vi "UHR-Fleezers Control (host) - 10.6.vi"() -> ()   [LabVIEW 2010] (continued)
    n794 = call <vilib>:"Mean.vi"("X"=w1127) -> ("mean"=w1106:dbl)  [unwired: 1 out]
    "T1 X" <- w1106
    n795 = Add(x=w1128, y=w1129) -> (x+y=w1130:dbl[])
    n796 = Bundle By Name(cluster=w1162, "Y"=w1124) -> (w1092:waveform(dbl))
    "Bead Separation" <- w1092
    n797 = Divide(x=w1130, y=2.0) -> (x/y=→"Vec Mean of T1 T2":dbl[])
    n798 = case shown="True" w1139 {
      tunnel: w1181 -> [_ w2041]
      tunnel: w1180 -> [_ w2040]
      tunnel: w1179 -> [_ w2039]
      tunnel: w1176 -> [_ w2038]
      tunnel: w1101 -> [_ w2037]
      frame False {
      }
      frame True {
        n799 = property on="Force" class="WFChart (strict)"("YScale.NameLbl.Text"=w2041) -> ()  [unwired: 2 in, 2 out]
        n800 = property on="T2 X" class="DigNum (strict)"("Caption.Text"=w2039) -> ()  [unwired: 2 in, 2 out]
        n801 = property on="T1 X" class="DigNum (strict)"("Caption.Text"=w2040) -> ()  [unwired: 2 in, 2 out]
        n802 = property on="Mean" class="DigNum (strict)"("Caption.Text"=w2038) -> ()  [unwired: 2 in, 2 out]
        n803 = property on="Difference" class="DigNum (strict)"("Caption.Text"=w2037) -> ()  [unwired: 2 in, 2 out]
      }
    }
    n804 = local read "Tether"() -> (w1133:bool)
    n805 = Absolute Value(x=w1106) -> (abs(x)=w1103:dbl)
    n806 = Absolute Value(x=w1105) -> (abs(x)=w1102:dbl)
    n807 = Add(x=w1103, y=w1102) -> (x+y=w1178:dbl)
    n808 = Subtract(x=w1103, y=w1102) -> (x-y=→"Difference":dbl)
    n809 = feedback #18(w1124) -> (w1123:dbl[])
    n810 = Divide(x=w1178, y=2.0) -> (x/y=w1132:dbl)
    "Mean" <- w1132
    n811 = case shown="True" w1133 {
      tunnel: w1132 -> [_ w1582]
      frame False {
      }
      frame True {
        n812 = Greater?(x="Lost Tether Alarm Threshold (pN)", y=w1582) -> (0:w1580:bool)
        n813 = case shown="True" w1580 {
          frame False {
          }
          frame True {
            n814 = flat-sequence {
              frame #0 {
                # "stop only if saving"
                n815 = local read "Saving..."() -> (w1595:bool)
                n816 = And(x=w1595, y="TA Cancel Save?") -> (x .and. y?=w1594:bool)
                n817 = local write "Stop Saving"(w1594) -> ()
              }
              frame #1 {
                n818 = case shown="True" "TA Green Off?" {
                  frame False {
                  }
                  frame True {
                    w1598 = FALSE ("Fl. Triggered...")
                    n819 = local write "Fl. Triggered..."(w1598) -> ()
                    n820 = property on="Green Laser ON/Interlacing" class="Bool (strict)"("Val(Sgnl)"=w1598) -> ()  [unwired: 2 in, 2 out]
                  }
                }
              }
            }
            n821 = local read "Time tether formed"() -> (w1589:timestamp)
            n822 = Get Date/Time In Seconds() -> (seconds since 1Jan1904=w1590:timestamp)
            n823 = Subtract(x=w1590, y=w1589) -> (x-y=w1588:dbl)
            n824 = Number To Decimal String(number=w1588) -> (decimal integer string=w1585:string)  [unwired: 1 out]
            n825 = local read "Messages"() -> (w1592:string)
            n826 = call <vilib>:"Beep.vi"() -> ()  [unwired: 3 in, 9 out]
            n827 = Concatenate Strings("Lost tether (" ("Message to add"), w1585, " s)." ("string")) -> (w1587:string)
            n828 = local write "Tether"(FALSE ("Tether")) -> ()
            n829 = call "Update messages.vi"("Message to add"=w1587, "Old message string"=w1592) -> ("New message string"=w1591:string)
            n830 = local write "Messages"(w1591) -> ()
            n831 = property on="Trap Pos. FB ON" class="Bool (strict)"("Val(Sgnl)"=FALSE ("Value (Signaling)")) -> ()  [unwired: 2 in, 2 out]
          }
        }
      }
    }
    n832 = Build Array (concatenate)(w1124, w1123) -> (w1122:dbl[])
    n833 = Split 1D Array(array=w1122, index=w1004) -> (first subarray=w1118:dbl[])  [unwired: 1 out]
    n834 = feedback-in #18(w1118) -> ()
    n835 = call <vilib>:"Mean.vi"("X"=w1118) -> ("mean"=w1117:dbl)  [unwired: 1 out]
    "Bead Mean (nm)" <- w1117
    n836 = Subtract(x=w1118, y=w1117) -> (x-y=w1116:dbl[])
    n837 = Square(x=w1116) -> (x^2=w1115:dbl[])
    n838 = call <vilib>:"Mean.vi"("X"=w1115) -> ("mean"=w1114:dbl)  [unwired: 1 out]
    n839 = Square Root(x=w1114) -> (sqrt(x)=w1113:dbl)
    n840 = Multiply(x=10.0, y=w1113) -> (x*y=→"RMS (Ang)":dbl)
    n841 = xnode "Read/Write Control"("FPGA VI Reference In"=w1154, "error in"=w1153) -> ("FPGA VI Reference Out"=w1270:T20, "error out"=w1264:errorcluster, "AI2 Y Sum Set 1"=w1260:i16, "AI2 Y Sum Set 2"=w1259:i16, "AI1 X Set 1"=w1038:fxp<+/-,16,1>, "AI1 X Set 2"=w1037:fxp<+/-,16,1>, "Trap Pos FB Int Signal"=→"Trap Pos FB Int Signal":fxp<+/-,24,9>, "Trap Pos FB Int-Norm Signal"=→"Trap Pos FB Int-Norm Signal":fxp<+/-,16,1>, "Trap Pos FB Action"=w1031:i64, "Scanning"=→"AOD Scanning":bool, "Scan I"=→"AOD Scan I":u64, "Scanning MCL"=w1262:bool, "Scan I (MCL)"=→"MCL Scan I":u64, "Green FB Signals"=w1199:T38)  [unwired: 1 out]
    "MCL Scanning" <- w1262
    "Trap Pos FB Action" <- w1031
    n842 = local read "AI2 (V)"() -> (w1261:cluster{"Set 1":dbl, "Set 2":dbl})
    n843 = Bundle By Name(cluster=w1261, "Set 1"=w1260, "Set 2"=w1259) -> (w1257:cluster{"Set 1":dbl, "Set 2":dbl})
    n844 = Divide(x=w1031, y=327.67) -> (x/y=→"Action (%)":dbl)
    n845 = local read "Trap X (AI1)"() -> (w1051:T10)
    n846 = Divide(x=w1257, y=3276.7) -> (x/y=w1256:cluster{"Set 1":dbl, "Set 2":dbl})
    n847 = local write "AI2 (V)"(w1256) -> ()
    n848 = Bundle(cluster=w1051, "Trap 1"=w1038, "Trap 2"=w1037) -> (→"Trap X (AI1)":T10)
    n849 = Divide(x=w1199, y=3276.7) -> (x/y=w1195:T46)
    n850 = Unbundle By Name(w1195) -> ("Green FB Ch 0"=w1198:dbl, "Green FB Ch 1"=w1197:dbl, "Green FB Ch 2"=w1196:dbl)
    n851 = Divide(x=w1198, y=w1196) -> (x/y=w1194:dbl)
    n852 = Divide(x=w1197, y=w1196) -> (x/y=w1193:dbl)
    n853 = flat-sequence "To save data" {
      tunnel: [w3898] -> w1281
      tunnel: [w3899] -> w1280
      tunnel: w1230 -> [w3892]
      tunnel: w1120 -> [w3896]
      tunnel: ["Save Calibration"] -> w1253
      tunnel: w1250 -> [w3895]
      tunnel: [w3888] -> w1249
      tunnel: [w3885] -> w1248
      tunnel: [w3882] -> w1247
      tunnel: w1229 -> [w3884]
      tunnel: w1137 -> [w3878]
      tunnel: [w3878] -> w1136
      tunnel: ["Start Saving"] -> w1094
      tunnel: [w3872] -> w1020
      tunnel: [w3871] -> w1019
      tunnel: w1281 -> [w4133]
      tunnel: w1280 -> [w4132]
      tunnel: w1021 -> [w4131]
      tunnel: w1253 -> [w4130]
      tunnel: w1249 -> [w4128]
      tunnel: w1248 -> [w4127]
      tunnel: w1247 -> [w4126]
      tunnel: w1107 -> [w4125]
      tunnel: w1146 -> [w4124]
      tunnel: w1136 -> [w4123]
      tunnel: w1094 -> [w4122]
      tunnel: w1092 -> [w4121]
      tunnel: w1068 -> [w4120]
      tunnel: w1020 -> [w4119]
      tunnel: w1019 -> [w4118]
      tunnel: w1018 -> [w4117]
      frame #0 {
        n854 = Or(x="Save N Sets", y="Start Saving") -> (x .or. y?=w3879:bool)
        n855 = To Double Precision Float(number=w3895) -> (double precision float=w3889:dbl)
        n856 = Build Array(w3879, "Save Calibration", w3892, w3884) -> (w3894:bool[])
        n857 = Compound Arithmetic op=OR("Save Calibration", w3892, w3879, w3884) -> (w3897:bool)
        n858 = Boolean Array To Number(Boolean array=w3894) -> (number=w3891:u32)
        n859 = feedback #19(FALSE ("Save APD Data\nwith Trap Data")) -> (w3873:bool)
        n860 = feedback #20(refnum<k0> refnum) -> (w3900:refnum<file>)
        n861 = feedback #21(refnum<k0> refnum) -> (w3875:refnum<file>)
        n862 = feedback #22(FALSE ("Save APD Data\nwith Trap Data")) -> (w3883:bool)
        n863 = feedback #23(refnum<k0> refnum) -> (w3886:refnum<file>)
        n864 = feedback #24(0) -> (w3902:i32)
        n865 = feedback #25() -> (w3890:u32)  [unwired: 1 out]
        n866 = case shown="True" w3897 {
          tunnel: [w3909 1] -> w3898
          tunnel: w3902 -> [w3911 _]
          tunnel: [w3910 w3929] -> w3899
          tunnel: w3900 -> [w3910 _]
          tunnel: w3896 -> [_ w3949]
          tunnel: w3889 -> [_ w3947]
          tunnel: w3891 -> [_ w3950]
          tunnel: [w3908 w3928] -> w3888
          tunnel: w3890 -> [w3908 _]
          tunnel: [w3907 w3926] -> w3885
          tunnel: w3886 -> [w3907 _]
          tunnel: [w3906 w3925] -> w3882
          tunnel: w3883 -> [w3906 _]
          tunnel: "Start Saving" -> [_ w3923]
          tunnel: w3878 -> [_ w3922]
          tunnel: [w3905 w3913] -> w3871
          tunnel: w3875 -> [w3905 _]
          tunnel: [w3904 w3912] -> w3872
          tunnel: w3873 -> [w3904 _]
          frame False {
            n867 = Increment(x=w3911) -> (x+1=w3909:i32)
          }
          frame True {
            w3919 = FALSE ("Start Saving")
            w3924 = 9.0  # File Version
            w3932 = FALSE ("prepend array or string size? (T)")
            w3930 = T39."big-endian, network order" ("byte order (0:big-endian, network order)")
            # "write file headers"
            n868 = local read "BD 1 Frequency 1 (MHz)"() -> (w3946:dbl)
            n869 = local read "BD 2 Frequency 1 (MHz)"() -> (w3945:dbl)
            n870 = local read "BD 1 Frequency 2 (MHz)"() -> (w3944:dbl)
            n871 = local read "BD 2 Frequency 2 (MHz)"() -> (w3943:dbl)
            n872 = local read "BD 1 Frequency 3 (MHz)"() -> (w3942:dbl)
            n873 = local read "BD 2 Frequency 3 (MHz)"() -> (w3941:dbl)
            n874 = Array Size(array=w3922) -> (size(s)=w3921:i32)
            n875 = To Double Precision Float(number=w3921) -> (double precision float=w3920:dbl)
            n876 = local write "Save Calibration"(w3919) -> ()
            n877 = local write "Start Saving"(w3919) -> ()
            n878 = Build Array("Save APD Data\nwith Trap Data", "Save Trap Pos. Data") -> (w3916:bool[])
            n879 = Boolean Array To Number(Boolean array=w3916) -> (number=w3915:u32)
            n880 = Build Array(w3946, w3945, w3944, w3943, w3942, w3941) -> (w3940:dbl[])
            n881 = case shown="2" w3950 {
              tunnel: w3949 -> [w4021 w4041 w4057 w4095]
              tunnel: w3920 -> [w4026 w4048 w4077 w4114]
              tunnel: w3947 -> [w4025 w4047 w4076 w4113]
              tunnel: [w4022 w4043 w4068 w4105] -> w3938
              tunnel: [w4013 "Cal sets to save" w4058 w4096] -> w3928
              tunnel: w3940 -> [w4023 w4044 w4070 w4107]
              tunnel: "Save APD Data\nwith Trap Data" -> [w4020 _ w4054 w4093]
              tunnel: [w4020 w4035 w4054 w4093] -> w3925
              tunnel: w3924 -> [w4016 w4036 w4052 w4091]
              tunnel: w3923 -> [w4015 _ _ _]
              tunnel: [w4006 w4035 w4051 w4081] -> w3912
              tunnel: "Save Trap Pos. Data" -> [w4006 _ w4051 w4081]
              tunnel: w3915 -> [w4005 _ w4050 w4080]
              frame 1, Default {
                # "timeseries"
                n882 = case shown="True" "Profile" {
                  tunnel: [w4029 w4032] -> w4010
                  tunnel: [w4029 w4031] -> w4009
                  tunnel: [w4029 w4030] -> w4008
                  tunnel: [w4029 w4034] -> w4007
                  frame False {
                    w4029 = 0.0 ("f")
                  }
                  frame True {
                    n883 = local read "Current Position"() -> (w4033:dbl[])
                    n884 = local read "Y change (mm)"() -> (w4034:dbl)
                    n885 = call "subVI_explode3array.vi"("Array"=w4033) -> ("x"=w4032:dbl, "y"=w4031:dbl, "z"=w4030:dbl)  [unwired: 12 in]
                  }
                }
                n886 = local read "Save ave N"() -> (w4028:dbl)
                n887 = Multiply(x=w4028, y=w4021) -> (x*y=w4027:dbl)
                n888 = To Double Precision Float(number=w4005) -> (double precision float=w4019:dbl)
                n889 = Build Array(w4016, w4021, w4027, w4026, w4025, 0.0 ("f")) -> (w4024:dbl[])
                n890 = Build Array(w4019, w4010, w4009, w4008, w4007) -> (w4017:dbl[])
                n891 = Select(t=u32 4000000000, s=w4015, f="N sets to save") -> (s? t:f=w4013:u32)
                n892 = Build Array (concatenate)(w4024, w4023, w4017) -> (w4022:dbl[])
              }
              frame 2 {
                w4038 = 0.0 ("f")
                w4035 = FALSE ("Save APD Data\nwith Trap Data")
                # "calibration"
                n893 = Boolean To (0,1)(Boolean=w4035) -> (0, 1=w4040:i16)
                n894 = To Double Precision Float(number=w4040) -> (double precision float=w4039:dbl)
                n895 = Build Array(w4039, w4038, w4038, w4038, w4038) -> (w4037:dbl[])
                n896 = Build Array(w4036, w4041, w4041, w4048, w4047, 1.0 ("t")) -> (w4045:dbl[])
                n897 = Build Array (concatenate)(w4045, w4044, w4037) -> (w4043:dbl[])
                "Calibrating Trap..." <- TRUE ("Calibrating...")
              }
              frame 4 {
                w4055 = 0.0 ("f")
                # "scan dir (x/y = 0/1)"
                # "cycles/step"
                # "n scans (f/b)"
                # "steps"
                # "freq. range"
                # "AOD raster scan"
                n898 = local read "Number of F/B Scans (AOD)"() -> (w4062:u16)
                n899 = local read "Cycles/step (AOD)"() -> (w4064:u64)
                n900 = local read "Scan Range (MHz)"() -> (w4067:dbl)
                n901 = local read "Scan steps (AOD)"() -> (w4066:u64)
                n902 = local read "Scan BD"() -> (w4074:bool)
                n903 = local read "Save ave N"() -> (w4079:dbl)
                n904 = Boolean To (0,1)(Boolean=w4074) -> (0, 1=w4073:i16)
                n905 = To Double Precision Float(number=w4062) -> (double precision float=w4061:dbl)
                n906 = To Double Precision Float(number=w4066) -> (double precision float=w4065:dbl)
                n907 = To Double Precision Float(number=w4064) -> (double precision float=w4063:dbl)
                n908 = To Double Precision Float(number=w4073) -> (double precision float=w4072:dbl)
                n909 = Multiply(x=w4079, y=w4057) -> (x*y=w4078:dbl)
                n910 = To Double Precision Float(number=w4050) -> (double precision float=w4056:dbl)
                n911 = Build Array(w4056, w4055, w4055, w4055, w4055) -> (w4053:dbl[])
                n912 = local read "N sets should be saved"() -> (w4059:dbl)
                n913 = Build Array(w4072, w4067, w4065, w4063, w4061) -> (w4069:dbl[])
                n914 = Build Array(w4052, w4057, w4078, w4077, w4076, 2.0 ("t")) -> (w4071:dbl[])
                n915 = Round Toward +Infinity(x=w4059) -> (ceil(x): smallest int >= x=w4060:dbl)
                n916 = Build Array (concatenate)(w4071, w4070, w4053, w4069) -> (w4068:dbl[])
                n917 = To Unsigned Long Integer(number=w4060) -> (unsigned 32bit integer=w4058:u32)
              }
              frame 8 {
                w4088 = 0.0 ("f")
                # "MCL raster scan"
                n918 = local read "Number of scans (MCL)"() -> (w4083:u64)
                n919 = local read "Scan lines (y)"() -> (w4082:u64)
                n920 = local read "2D or 1D Scan"() -> (w4085:bool)
                n921 = local read "Scan Range (V)\n(of steps)"() -> (w4104:dbl)
                n922 = local read "Fast Scan Dir"() -> (w4111:bool)
                n923 = local read "Cycles/step (MCL)"() -> (w4101:u64)
                n924 = local read "Scan steps (MCL)"() -> (w4103:u64)
                n925 = Select(t=w4082, s=w4085, f=w4083) -> (s? t:f=w4084:u64)
                n926 = Boolean To (0,1)(Boolean=w4085) -> (0, 1=w4087:i16)
                n927 = local read "Save ave N"() -> (w4116:dbl)
                n928 = local read "Initial X"() -> (w4090:dbl)
                n929 = local read "Initial Y"() -> (w4089:dbl)
                n930 = To Double Precision Float(number=w4087) -> (double precision float=w4086:dbl)
                n931 = Boolean To (0,1)(Boolean=w4111) -> (0, 1=w4110:i16)
                n932 = To Double Precision Float(number=w4084) -> (double precision float=w4099:dbl)
                n933 = To Double Precision Float(number=w4103) -> (double precision float=w4102:dbl)
                n934 = To Double Precision Float(number=w4101) -> (double precision float=w4100:dbl)
                n935 = To Double Precision Float(number=w4110) -> (double precision float=w4109:dbl)
                n936 = Multiply(x=w4116, y=w4095) -> (x*y=w4115:dbl)
                n937 = To Double Precision Float(number=w4080) -> (double precision float=w4094:dbl)
                n938 = local read "N sets should be saved (MCL)"() -> (w4097:dbl)
                n939 = Build Array(w4094, w4086, w4088, w4088, w4088) -> (w4092:dbl[])
                n940 = Build Array(w4109, w4104, w4102, w4100, w4099, w4090, w4089) -> (w4106:dbl[])
                n941 = Build Array(w4091, w4095, w4115, w4114, w4113, 3.0 ("t")) -> (w4108:dbl[])
                n942 = Round Toward +Infinity(x=w4097) -> (ceil(x): smallest int >= x=w4098:dbl)
                n943 = Build Array (concatenate)(w4108, w4107, w4092, w4106) -> (w4105:dbl[])
                n944 = To Unsigned Long Integer(number=w4098) -> (unsigned 32bit integer=w4096:u32)
              }
            }
            n945 = local read "Index"() -> (w3955:dbl)
            n946 = call "Create new save file.vi"("Insert"="", "Ext"=".dat", "Index In"=w3955) -> ("Path Out"=w3914:path, "Index Out"=w3927:dbl)
            n947 = local write "Save file name"(w3914) -> ()
            n948 = local write "Index"(w3927) -> ()
            n949 = local write "Save index"(w3927) -> ()
            n950 = Array Size(array=w3938) -> (size(s)=w3939:i32)
            n951 = Open/Create/Replace File(file path (use dialog)=w3914, operation (0:open)=T25."create", access (0:read/write)=enum16{"read/write", "read-only", "write-only"}."write-only") -> (refnum out=w3952:refnum<file>)  [unwired: 1 in, 4 out]
            n952 = local write "Saving..."(TRUE ("Saving...")) -> ()
            n953 = To Double Precision Float(number=w3939) -> (double precision float=w3937:dbl)
            n954 = String Length(string="Comment (data description)") -> (length=w3935:i32)
            n955 = To Double Precision Float(number=w3935) -> (double precision float=w3934:dbl)
            n956 = Deny Access(7:w3952) -> (3:w3951:refnum<file>)  [unwired: 1 in, 2 out]
            n957 = Build Array (concatenate)(w3937, w3938, w3934) -> (w3936:dbl[])
            n958 = case "If fluorescence data to be saved" shown="False" w3925 {
              tunnel: w3914 -> [_ w4004]
              tunnel: [refnum<k0> refnum w3984] -> w3926
              frame False {
              }
              frame True {
                w3983 = 0.0
                n959 = local read "APD Integration Time (s)"() -> (w3989:dbl)
                n960 = local read "N APD Samp/step"() -> (w3982:dbl)
                n961 = Path To String(path=w4004) -> (string=w4003:string)
                n962 = String Length(string=w4003) -> (length=w4002:i32)
                n963 = Subtract(x=w4002, y=4) -> (x-y=w4000:i32)
                n964 = String Subset(string=w4003, length (rest)=w4000) -> (substring=w3999:string)  [unwired: 1 out]
                n965 = Build Array(w3989, w3982, w3983, w3983, w3983, w3983, w3983, w3983) -> (w3986:dbl[])
                n966 = Concatenate Strings(w3999, "_fl.dat" ("string")) -> (w3997:string)
                n967 = Array Size(array=w3986) -> (size(s)=w3988:i32)
                n968 = String To Path(string=w3997) -> (path=w3993:path)
                n969 = Open/Create/Replace File(file path (use dialog)=w3993, operation (0:open)=T25."create", access (0:read/write)=enum16{"read/write", "read-only", "write-only"}."write-only") -> (refnum out=w3994:refnum<file>)  [unwired: 1 in, 4 out]
                n970 = Deny Access(7:w3994) -> (3:w3990:refnum<file>)  [unwired: 1 in, 2 out]
                n971 = To Double Precision Float(number=w3988) -> (double precision float=w3987:dbl)
                n972 = Build Array (concatenate)(w3987, w3986) -> (w3985:dbl[])
                n973 = Write to Binary File(file (use dialog)=w3990, data=w3985, 5:FALSE ("prepend array or string size? (T)"), 9:T39."big-endian, network order" ("byte order (0:big-endian, network order)")) -> (refnum out=w3984:refnum<file>)  [unwired: 1 in, 3 out]
              }
            }
            n974 = case shown="True" w3912 {
              tunnel: w3914 -> [_ w3966]
              tunnel: [refnum<k0> refnum w3965] -> w3913
              frame False {
              }
              frame True {
                w3961 = 0.0 ("element")
                n975 = Path To String(path=w3966) -> (string=w3980:string)
                n976 = Build Array(w3961, w3961, w3961, w3961, w3961, w3961, w3961, w3961) -> (w3962:dbl[])
                n977 = String Length(string=w3980) -> (length=w3979:i32)
                n978 = Subtract(x=w3979, y=4) -> (x-y=w3977:i32)
                n979 = Array Size(array=w3962) -> (size(s)=w3964:i32)
                n980 = String Subset(string=w3980, length (rest)=w3977) -> (substring=w3976:string)  [unwired: 1 out]
                n981 = To Double Precision Float(number=w3964) -> (double precision float=w3963:dbl)
                n982 = Concatenate Strings(w3976, "_pos.dat" ("string")) -> (w3974:string)
                n983 = Build Array (concatenate)(w3963, w3962) -> (w3960:dbl[])
                n984 = String To Path(string=w3974) -> (path=w3970:path)
                n985 = Open/Create/Replace File(file path (use dialog)=w3970, operation (0:open)=T25."create", access (0:read/write)=enum16{"read/write", "read-only", "write-only"}."write-only") -> (refnum out=w3971:refnum<file>)  [unwired: 1 in, 4 out]
                n986 = Deny Access(7:w3971) -> (3:w3967:refnum<file>)  [unwired: 1 in, 2 out]
                n987 = Write to Binary File(file (use dialog)=w3967, data=w3960, 5:FALSE ("prepend array or string size? (T)"), 9:T39."big-endian, network order" ("byte order (0:big-endian, network order)")) -> (refnum out=w3965:refnum<file>)  [unwired: 1 in, 3 out]
              }
            }
            n988 = Write to Binary File(file (use dialog)=w3951, data=w3936, 5:w3932, 9:w3930) -> (refnum out=w3933:refnum<file>)  [unwired: 1 in, 3 out]
            n989 = Write to Binary File(file (use dialog)=w3933, data="Comment (data description)", 5:w3932, 9:w3930) -> (refnum out=w3929:refnum<file>)  [unwired: 1 in, 3 out]
          }
        }
        n990 = feedback-in #19(w3872) -> ()
        n991 = feedback-in #20(w3899) -> ()
        n992 = feedback-in #21(w3871) -> ()
        n993 = feedback-in #22(w3882) -> ()
        n994 = feedback-in #23(w3885) -> ()
        n995 = feedback-in #24(w3898) -> ()
        n996 = feedback-in #25(w3888) -> ()
      }
      frame #1 {
        n997 = local read "Saving..."() -> (w4129:bool)
        n998 = case shown="True" w4129 {
          tunnel: w4133 -> [_ w4143]
          tunnel: w4132 -> [_ w4157]
          tunnel: w4131 -> [_ w4153]
          tunnel: w4130 -> [_ w4152]
          tunnel: w4128 -> [_ w4151]
          tunnel: w4127 -> [_ w4146]
          tunnel: w4126 -> [_ w4145]
          tunnel: w4125 -> [_ w4144]
          tunnel: w4124 -> [_ w4142]
          tunnel: w4123 -> [_ w4140]
          tunnel: w4122 -> [_ w4139]
          tunnel: w4121 -> [_ w4138]
          tunnel: w4120 -> [_ w4137]
          tunnel: w4119 -> [_ w4136]
          tunnel: w4118 -> [_ w4135]
          tunnel: w4117 -> [_ w4134]
          frame False {
          }
          frame True {
            n999 = Multiply(x=w4143, y=w4142) -> (x*y=→"Time (s)":dbl)
            n1000 = Less Or Equal?(x=w4143, y=w4151) -> (x <= y?=w4155:bool)
            n1001 = Or(x="Stop Saving", y="Abort save 2") -> (x .or. y?=w4147:bool)
            n1002 = Not(x=w4147) -> (.not. x?=w4156:bool)
            n1003 = And(x=w4155, y=w4156) -> (x .and. y?=w4154:bool)
            n1004 = case shown="True" w4154 {
              tunnel: w4157 -> [w4164 w4232]
              tunnel: [0.0 w4235] -> w4150
              tunnel: w4143 -> [_ w4233]
              tunnel: w4151 -> [_ w4234]
              tunnel: w4153 -> [_ w4229]
              tunnel: w4152 -> [_ _]
              tunnel: w4146 -> [w4162 w4222]
              tunnel: w4145 -> [w4161 w4223]
              tunnel: w4144 -> [_ w4221]
              tunnel: w4140 -> [_ w4220]
              tunnel: w4139 -> [_ w4174]
              tunnel: w4138 -> [_ w4213]
              tunnel: w4137 -> [_ w4191]
              tunnel: w4136 -> [w4158 w4172]
              tunnel: w4135 -> [w4159 w4171]
              tunnel: w4134 -> [_ w4168]
              frame False {
                w4160 = FALSE
                n1005 = Close File(refnum=w4164) -> ()  [unwired: 1 in, 2 out]
                n1006 = case shown="True" w4161 {
                  tunnel: w4162 -> [_ w4166]
                  frame False {
                  }
                  frame True {
                    n1007 = Close File(refnum=w4166) -> ()  [unwired: 1 in, 2 out]
                  }
                }
                n1008 = case shown="True" w4158 {
                  tunnel: w4159 -> [_ w4165]
                  frame False {
                  }
                  frame True {
                    n1009 = Close File(refnum=w4165) -> ()  [unwired: 1 in, 2 out]
                  }
                }
                n1010 = local write "Raster Scanning..."(w4160) -> ()
                n1011 = local write "Calibrating Trap..."(w4160) -> ()
                n1012 = call <vilib>:"Beep.vi"() -> ()  [unwired: 3 in, 9 out]
                n1013 = local write "Stop Saving"(w4160) -> ()
                "Saving..." <- w4160
              }
              frame True {
                n1014 = local read "Calibrating Trap..."() -> (w4224:bool)
                n1015 = case "Write fl. data" shown="True" w4223 {
                  tunnel: w4222 -> [_ w4258]
                  tunnel: w4221 -> [_ w4257]
                  frame False {
                  }
                  frame True {
                    n1016 = Write to Binary File(file (use dialog)=w4258, data=w4257, 5:FALSE ("prepend array or string size? (T)"), 9:T39."big-endian, network order" ("byte order (0:big-endian, network order)")) -> ()  [unwired: 1 in, 4 out]
                  }
                }
                n1017 = Greater?(x="Save ave N", y=1.0) -> (0:w4227:bool)
                n1018 = Not(x=w4224) -> (.not. x?=w4226:bool)
                n1019 = And(x=w4226, y=w4227) -> (x .and. y?=w4169:bool)
                n1020 = case shown="True" w4169 {
                  tunnel: w4168 -> [w4238 w4249]
                  tunnel: [w4238 w4241] -> w4167
                  tunnel: "Save ave N" -> [_ w4242]
                  frame False {
                  }
                  frame True {
                    w4239 = 2 ("dimension size")
                    n1021 = Array Size(array=w4249) -> (size(s)=w4243:i32)
                    n1022 = Divide(x=w4243, y=w4239) -> (x/y=w4247:dbl)
                    n1023 = Reshape Array(w4249, w4247, w4239) -> (w4248:u64[][])
                    n1024 = Transpose 2D Array(2D array=w4248) -> (transposed array=w4246:u64[][])
                    n1025 = for {
                      tunnel: w4246 -> [w4251] mode=indexing
                      tunnel: [w4250] -> w4240 mode=indexing
                      tunnel: w4242 -> [w4252]
                      workers-P: _ -> [_]
                      n1026 = call "downsample 1D array - U64.vi"("Ave N"=w4252, "Array In"=w4251) -> ("Array Out"=w4250:u64[])  [unwired: 1 in]
                    }
                    n1027 = Transpose 2D Array(2D array=w4240) -> (transposed array=w4245:u64[][])
                    n1028 = Divide(x=w4243, y=w4242) -> (x/y=w4244:dbl)
                    n1029 = Reshape Array(w4245, w4244) -> (w4241:u64[])
                  }
                }
                n1030 = case shown="True" w4169 {
                  tunnel: w4229 -> [w4261 w4273]
                  tunnel: [w4261 w4262] -> w4225
                  tunnel: "Save ave N" -> [_ w4266]
                  tunnel: w4220 -> [_ w4265]
                  frame False {
                    # "don't downsample data for trap calibration"
                  }
                  frame True {
                    n1031 = Array Size(array=w4273) -> (size(s)=w4267:i32)
                    n1032 = Array Size(array=w4265) -> (size(s)=w4264:i32)
                    n1033 = Divide(x=w4267, y=w4264) -> (x/y=w4271:dbl)
                    n1034 = Reshape Array(w4273, w4271, w4264) -> (w4272:i16[][])
                    n1035 = Transpose 2D Array(2D array=w4272) -> (transposed array=w4270:i16[][])
                    n1036 = for {
                      tunnel: w4270 -> [w4276] mode=indexing
                      tunnel: [w4275] -> w4263 mode=indexing
                      tunnel: w4266 -> [w4274]
                      workers-P: _ -> [_]
                      n1037 = call "downsample 1D array - I16.vi"("Ave N"=w4274, "Array In"=w4276) -> ("Array Out"=w4275:i16[])  [unwired: 1 out]
                    }
                    n1038 = Transpose 2D Array(2D array=w4263) -> (transposed array=w4269:i16[][])
                    n1039 = Divide(x=w4267, y=w4266) -> (x/y=w4268:dbl)
                    n1040 = Reshape Array(w4269, w4268) -> (w4262:i16[])
                  }
                }
                n1041 = Index Array(array=w4191, index=1) -> (element=w4194:waveform(dbl))
                n1042 = Index Array(array=w4191, index=0) -> (element=w4196:waveform(dbl))
                n1043 = Unbundle By Name(w4194) -> ("Y"=w4198:dbl[])
                n1044 = Unbundle By Name(w4196) -> ("Y"=w4206:dbl[])
                n1045 = case "Write trap pos. data" shown="True" w4172 {
                  tunnel: w4171 -> [_ w4254]
                  tunnel: w4167 -> [_ w4253]
                  frame False {
                  }
                  frame True {
                    n1046 = Write to Binary File(file (use dialog)=w4254, data=w4253, 5:FALSE ("prepend array or string size? (T)"), 9:T39."big-endian, network order" ("byte order (0:big-endian, network order)")) -> ()  [unwired: 1 in, 4 out]
                  }
                }
                n1047 = Write to Binary File(file (use dialog)=w4232, data=w4225, 5:FALSE ("prepend array or string size? (T)"), 9:T39."big-endian, network order" ("byte order (0:big-endian, network order)")) -> ()  [unwired: 1 in, 4 out]
                n1048 = feedback #26(w4198) -> (w4200:dbl[])
                n1049 = Build Array (concatenate)(w4200, w4198) -> (w4199:dbl[])
                n1050 = Select(t=w4198, s=w4174, f=w4199) -> (s? t:f=w4184:dbl[])
                n1051 = feedback-in #26(w4184) -> ()
                n1052 = feedback #27(w4206) -> (w4219:dbl[])
                n1053 = Build Array (concatenate)(w4219, w4206) -> (w4218:dbl[])
                n1054 = Select(t=w4206, s=w4174, f=w4218) -> (s? t:f=w4193:dbl[])
                n1055 = feedback-in #27(w4193) -> ()
                n1056 = Divide(x=w4233, y=w4234) -> (x/y=w4236:dbl)
                n1057 = Multiply(x=w4236, y=100.0) -> (x*y=w4235:dbl)
                n1058 = Build Array(w4193, w4184) -> (→"Saved APD":dbl[][])
                n1059 = Array Size(array=w4193) -> (size(s)=w4211:i32)
                n1060 = Unbundle By Name(w4213) -> ("Y"=w4217:dbl[])
                n1061 = Subtract(x=w4211, y="N pts to average") -> (x-y=w4187:i32)
                n1062 = Multiply(x="N pts to average", y=u16 2) -> (x*y=w4188:u16)
                n1063 = Subtract(x=w4211, y=w4188) -> (x-y=w4186:i32)
                n1064 = feedback #28(w4217) -> (w4216:dbl[])
                n1065 = Build Array (concatenate)(w4216, w4217) -> (w4215:dbl[])
                n1066 = Select(t=w4217, s=w4174, f=w4215) -> (s? t:f=w4214:dbl[])
                "Trap Delta Graph" <- w4214
                n1067 = feedback-in #28(w4214) -> ()
                n1068 = Array Subset(array=w4193, index=w4187, length="N pts to average") -> (w4210:dbl[])
                n1069 = Array Subset(array=w4193, index=w4186, length="N pts to average") -> (w4209:dbl[])
                n1070 = Array Subset(array=w4184, index=w4187, length="N pts to average") -> (w4190:dbl[])
                n1071 = Array Subset(array=w4184, index=w4186, length="N pts to average") -> (w4189:dbl[])
                n1072 = call <vilib>:"Mean.vi"("X"=w4210) -> ("mean"=w4208:dbl)  [unwired: 1 out]
                n1073 = call <vilib>:"Mean.vi"("X"=w4190) -> ("mean"=w4183:dbl)  [unwired: 1 out]
                n1074 = call <vilib>:"Mean.vi"("X"=w4209) -> ("mean"=w4207:dbl)  [unwired: 1 out]
                n1075 = call <vilib>:"Mean.vi"("X"=w4189) -> ("mean"=w4182:dbl)  [unwired: 1 out]
                n1076 = Subtract(x=w4183, y=w4182) -> (x-y=w4173:dbl)
                "Delta Fl. 2" <- w4173
                n1077 = Subtract(x=w4208, y=w4207) -> (x-y=w4205:dbl)
                "Delta Fl. 1" <- w4205
                n1078 = Initialize Array(w4205, 1 ("dimension size")) -> (w4202:dbl[])
                n1079 = Initialize Array(w4173, 1 ("dimension size")) -> (w4179:dbl[])
                n1080 = feedback #29(w4202) -> (w4203:dbl[])
                n1081 = Build Array (concatenate)(w4203, w4202) -> (w4201:dbl[])
                n1082 = feedback #30(w4179) -> (w4180:dbl[])
                n1083 = Build Array (concatenate)(w4180, w4179) -> (w4178:dbl[])
                n1084 = Select(t=w4202, s=w4174, f=w4201) -> (s? t:f=w4177:dbl[])
                n1085 = feedback-in #29(w4177) -> ()
                n1086 = Select(t=w4179, s=w4174, f=w4178) -> (s? t:f=w4176:dbl[])
                n1087 = feedback-in #30(w4176) -> ()
                n1088 = Build Array(w4177, w4176) -> (→"Save APD Deriv":dbl[][])
              }
            }
            "Progress" <- w4150
            "Progress 2" <- w4150
          }
        }
      }
    }
    n1089 = Bundle By Name(cluster=w1195, "Green FB Ch 0"=w1194, "Green FB Ch 1"=w1193) -> (w1175:T46)
    "Green FB Signals (V)" <- w1175
    n1090 = Unbundle By Name(w1175) -> ("Green FB Ch 2"=→"Green FB Plot":dbl)
    n1091 = local read "wait to reset values"() -> (w1265:bool)
    n1092 = Not(x=w1262) -> (.not. x?=w1266:bool)
    n1093 = And(x=w1266, y=w1265) -> (x .and. y?=w1267:bool)
    n1094 = case "Part of MCL raster scanning: returns to initial positions after scan done" shown="True" w1267 {
      tunnel: w1270 -> [w2867 w2874]
      tunnel: [w2867 w2873] -> w1269
      tunnel: w1264 -> [w2866 w2872]
      tunnel: [w2866 w2871] -> w1263
      frame False {
      }
      frame True {
        w2882 = 10.0 ("y")
        w2881 = 32767.0 ("y")
        # "to return scan values\nafter a synchronous \nAOM scan"
        n1095 = local read "AO2"() -> (w2875:dbl)
        n1096 = local read "AO1"() -> (w2876:dbl)
        n1097 = local write "wait to reset values"(FALSE ("wait to reset values")) -> ()
        n1098 = Multiply(x=w2876, y=w2881) -> (x*y=w2878:dbl)
        n1099 = Multiply(x=w2875, y=w2881) -> (x*y=w2880:dbl)
        n1100 = Divide(x=w2878, y=w2882) -> (x/y=w2877:dbl)
        n1101 = Divide(x=w2880, y=w2882) -> (x/y=w2879:dbl)
        n1102 = To Word Integer(number=w2877) -> (16bit integer=w2883:i16)
        n1103 = To Word Integer(number=w2879) -> (16bit integer=w2884:i16)
        n1104 = local read "Total Counts (ticks)"() -> (w2868:u32)
        n1105 = xnode "Read/Write Control"("FPGA VI Reference In"=w2874, "error in"=w2872, "AO1"=w2883, "AO2"=w2884, "MCL count"=w2868) -> ("FPGA VI Reference Out"=w2873:T20, "error out"=w2871:errorcluster)
        n1106 = local read "Scan Range (V)\n(of steps)"() -> (w2869:dbl)
        n1107 = property on="Scan Range (V)\n(of steps)" class="DigNum (strict)"("Val(Sgnl)"=w2869) -> ()  [unwired: 2 in, 2 out]
      }
    }
    n1108 = node-c288() -> ()  [unwired: 2 out]
  }
  n1109 = node-c288(3 ("Processor")) -> (w79:T26)  [unwired: 3 out]
  n1110 = disable-structure shown="Enabled" {
    disable-tunnel: [w4278 _] -> w34
    disable-tunnel: w18 -> [w4277 _]
    frame Enabled {
      n1111 = node-c288() -> (w4280:T26)  [unwired: 4 out]
      n1112 = timed-loop "Rough control of MCL mirror stage (debugging)" {
        tunnel: w4277 -> [w4283]
        tunnel: [w4282] -> w4278
        timing: w4280 -> [_]
        timing-out: [_] -> w4279
        stop <- w4282 stop-if-true
        n1113 = node-c288() -> ()  [unwired: 2 out]
        n1114 = case shown="1" "MCL Mode" {
          tunnel: w4283 -> [_ w4286 w4390]
          frame 0, Default {
            # "manual positioning"
          }
          frame 1 {
            # "sinusoidal wave"
            n1115 = node-c288() -> (w4288:T26)  [unwired: 4 out]
            n1116 = timed-loop "Oscillate MCL mirror" {
              timing: w4288 -> [_]
              timing-out: [_] -> w4287
              tunnel: w4286 -> [w4327]
              i -> [w4326]
              stop <- w4289 stop-if-true
              n1117 = node-c288() -> (w4325:i64)  [unwired: 1 out]
              n1118 = Multiply(x="AO1", y=32767.0) -> (x*y=w4321:dbl)
              n1119 = Multiply(x="AO2", y=32767.0) -> (x*y=w4316:dbl)
              n1120 = Divide(x=w4321, y=10.0) -> (x/y=w4322:dbl)
              n1121 = Divide(x=w4316, y=10.0) -> (x/y=w4317:dbl)
              n1122 = To Word Integer(number=w4322) -> (16bit integer=w4314:i16)
              n1123 = To Word Integer(number=w4317) -> (16bit integer=w4313:i16)
              n1124 = Divide(x=w4325, y=i64 1000) -> (x/y=w4296:dbl)
              n1125 = Multiply(x=w4296, y=w4326) -> (x*y=w4307:dbl)
              n1126 = Multiply(x="Osc. freq. (Hz) 2", y=6.283185307179586) -> (x*y=w4308:dbl)
              n1127 = Multiply(x=w4308, y=w4307) -> (x*y=w4306:dbl)
              n1128 = Sine(x=w4306) -> (sin(x)=w4305:dbl)
              n1129 = Multiply(x=w4305, y="Osc. amp. (V)") -> (x*y=w4303:dbl)
              n1130 = Add(x=w4303, y="Osc. center (V)") -> (x+y=w4301:dbl)
              n1131 = Divide(x=w4301, y=10.0) -> (x/y=w4299:dbl)
              n1132 = Multiply(x=w4299, y=32767.0) -> (x*y=w4294:dbl)
              n1133 = Select(t=w4294, s="Scan axis", f=w4314) -> (s? t:f=w4312:dbl)
              n1134 = Select(t=w4313, s="Scan axis", f=w4294) -> (s? t:f=w4311:dbl)
              n1135 = local read "MCL Mode"() -> (w4293:u16)
              n1136 = Not Equal?(x=w4293, y=u16 1) -> (x != y?=w4290:bool)
              n1137 = local read "Stop All"() -> (w4291:bool)
              n1138 = xnode "Read/Write Control"("FPGA VI Reference In"=w4327, "AO1"=w4312, "AO2"=w4311) -> ()  [unwired: 1 in, 2 out]
              n1139 = Compound Arithmetic op=OR(w4291, w4290) -> (w4289:bool)
              n1140 = node-c288() -> ()  [unwired: 2 out]
            }
            n1141 = node-c288(w4287) -> ()  [unwired: 1 out]
          }
          frame 2 {
            # "linear scan"
            n1142 = case shown="True" "Start Scan" {
              tunnel: w4390 -> [_ w4402]
              frame False {
              }
              frame True {
                n1143 = Subtract(x="End (V)", y="Begin (V)") -> (x-y=w4398:dbl)
                n1144 = Decrement(x="N Points") -> (x-1=w4397:dbl)
                n1145 = Divide(x=w4398, y=w4397) -> (x/y=w4395:dbl)
                n1146 = for {
                  N: "N Points" -> [_]
                  tunnel: "Begin (V)" -> [w4415]
                  tunnel: w4402 -> [w4407]
                  tunnel: [w4406] -> w4401 mode=indexing
                  tunnel: w4395 -> [w4405]
                  tunnel: [w4403] -> w4394 mode=indexing
                  i -> [w4414]
                  n1147 = Multiply(x=w4405, y=w4414) -> (x*y=w4413:dbl)
                  n1148 = Add(x=w4415, y=w4413) -> (x+y=w4410:dbl)
                  n1149 = local read "Scan axis"() -> (w4404:bool)
                  n1150 = local read "AO1"() -> (w4412:dbl)
                  n1151 = local read "AO2"() -> (w4411:dbl)
                  n1152 = Select(t=w4410, s=w4404, f=w4412) -> (s? t:f=w4409:dbl)
                  n1153 = Select(t=w4411, s=w4404, f=w4410) -> (s? t:f=w4408:dbl)
                  n1154 = flat-sequence {
                    tunnel: w4409 -> [w4419]
                    tunnel: w4408 -> [w4418]
                    tunnel: w4407 -> [w4416]
                    tunnel: [w4486] -> w4406
                    tunnel: [w4485] -> w4403
                    frame #0 {
                      w4422 = 10.0 ("y")
                      w4417 = 32767.0 ("y")
                      n1155 = Multiply(x=w4419, y=w4417) -> (x*y=w4425:dbl)
                      n1156 = Multiply(x=w4418, y=w4417) -> (x*y=w4423:dbl)
                      n1157 = Divide(x=w4425, y=w4422) -> (x/y=w4426:dbl)
                      n1158 = Divide(x=w4423, y=w4422) -> (x/y=w4424:dbl)
                      n1159 = To Word Integer(number=w4426) -> (16bit integer=w4420:i16)
                      n1160 = To Word Integer(number=w4424) -> (16bit integer=w4421:i16)
                      n1161 = xnode "Read/Write Control"("FPGA VI Reference In"=w4416, "AO1"=w4420, "AO2"=w4421) -> ()  [unwired: 1 in, 2 out]
                    }
                    frame #1 {
                      n1162 = Wait (ms)(milliseconds to wait="DAQ Delay (ms)") -> ()  [unwired: 1 out]
                    }
                    frame #2 {
                      n1163 = local read "Slow mean"() -> (w4486:dbl)
                      n1164 = local read "Sigma"() -> (w4485:dbl)
                    }
                  }
                }
                n1165 = Bundle("Begin (V)"="Begin (V)", w4395, w4401) -> (→"MCL Scan":cluster{"Begin (V)":dbl, dbl, dbl[]})  [unwired: 1 out]
                n1166 = Bundle("Begin (V)"="Begin (V)", w4395, w4394) -> (→"MCL Scan 2":cluster{"Begin (V)":dbl, dbl, dbl[]})  [unwired: 1 out]
              }
            }
          }
        }
        n1167 = local read "Stop All"() -> (w4282:bool)
        n1168 = node-c288() -> ()  [unwired: 2 out]
      }
      n1169 = node-c288(w4279) -> ()  [unwired: 1 out]
    }
    frame Disabled {
    }
  }
  n1170 = timed-loop "Control parameters (event loop)" {
    tunnel: w18 -> [w4493]
    shift-right: [w4492] -> w2
    shift-left: errorcluster {"status"=FALSE, "code"=0, "source"=""} ("error out") -> [w4491]
    tunnel: [w4490] -> w36
    tunnel: w60 -> [w4489]
    timing: w9 -> [_]
    timing-out: [_] -> w8
    stop <- w4490 stop-if-true
    n1171 = node-c288() -> ()  [unwired: 1 in, 1 out]
    n1172 = event shown="[51] \"Trap Pos. FB Range\", \"Trap Pos. FB Gains\", \"Trap Pos. FB Mult Factor\", \"Trap Pos. FB Offset Factor\", \"Trap Pos FB Negate Action\", \"Trap Pos FB Monitor\nT1 or T2\": Value Change" {
      selector: _ -> [_ _ _ _ _ _ _ _ _ _ _ _ _ _ _ _ _ _ _ _ _ _ _ _ _ _ _ _ _ _ _ _ _ _ _ _ _ _ _ _ _ _ _ _ _ _ _ _ _ _ _ _ _ _ _ _]
      dyn-events: _ -> [_ _ _ _ _ _ _ _ _ _ _ _ _ _ _ _ _ _ _ _ _ _ _ _ _ _ _ _ _ _ _ _ _ _ _ _ _ _ _ _ _ _ _ _ _ _ _ _ _ _ _ _ _ _ _ _]
      timeout: _ -> [_ _ _ _ _ _ _ _ _ _ _ _ _ _ _ _ _ _ _ _ _ _ _ _ _ _ _ _ _ _ _ _ _ _ _ _ _ _ _ _ _ _ _ _ _ _ _ _ _ _ _ _ _ _ _ _]
      tunnel: w4493 -> [w4531 _ _ _ w4653 _ w4750 _ w4814 _ _ _ w5008 _ _ w5110 w5254 w5318 w5393 w5547 w5624 w5755 _ w5851 w5937 w6023 w6109 w6195 w6281 w6374 w6538 w6749 w6892 w7029 _ _ w7303 w7345 w7393 w7472 w7514 _ w7560 _ _ _ _ w7765 _ w7858 w7899 w7946 w8134 w8183 _ w8245]
      tunnel: [w4530 _ _ _ w4643 _ w4749 _ w4777 _ w4973 _ w4987 _ _ w5109 w5250 w5315 w5390 w5546 w5622 w5754 _ w5845 w5931 w6017 w6103 w6189 w6275 w6372 w6537 w6747 w6890 w7027 _ _ w7301 w7343 w7383 w7470 w7512 _ w7558 w7628 w7677 w7725 w7752 w7763 _ _ _ _ _ _ _ _] -> w4492
      tunnel: w4491 -> [w4529 _ _ _ w4652 _ w4748 _ w4809 _ w4973 _ w5007 _ _ w5108 w5249 w5314 w5389 w5545 w5623 w5753 _ w5850 w5936 w6022 w6108 w6194 w6280 w6373 w6536 w6748 w6891 w7028 _ _ w7302 w7344 w7392 w7471 w7513 _ w7559 w7629 w7678 w7726 w7753 w7764 _ w7857 w7898 w7945 w8133 w8182 _ w8244]
      tunnel: [_ _ _ _ _ _ _ _ _ _ w4972 _ _ _ _ _ _ _ _ _ _ _ _ _ _ _ _ _ _ _ _ _ _ _ _ _ _ _ _ _ _ _ _ _ _ _ _ _ _ _ _ _ _ _ _ _] -> w4490
      tunnel: [_ _ _ _ _ _ _ "Round T1 X" _ _ _ _ _ _ _ _ _ _ _ _ _ _ _ _ _ _ _ _ _ _ _ _ _ _ _ _ _ _ _ _ _ _ _ _ _ _ _ _ _ _ _ _ _ _ _ _] -> _
      tunnel: [_ _ _ "Adjust Scale\nto Mean" _ _ _ _ _ _ _ _ _ _ _ _ _ _ _ _ _ _ _ _ _ _ _ _ _ _ _ _ _ _ _ _ _ _ _ _ _ _ _ _ _ _ _ _ _ _ _ _ _ "Set SP to Reading" _ _] -> _
      tunnel: [_ _ _ _ _ _ _ _ _ "Round T2 X" _ "Delayed Interlace Start" _ _ _ _ _ _ _ _ _ _ _ _ _ _ _ _ _ _ _ _ _ _ _ _ _ _ _ _ _ _ _ _ _ _ _ _ _ _ _ _ _ _ _ _] -> _
      tunnel: w4489 -> [_ _ _ _ _ _ _ _ _ _ _ _ _ _ _ _ _ _ _ _ _ _ _ _ _ _ _ _ _ _ _ _ _ _ _ _ _ _ _ _ _ _ _ _ _ _ _ _ _ _ _ _ _ _ _ _]
      event "AI Count (ticks)", "Sets to FIFO (Traps)", "Save ave N", "FPGA Ave.", "# Samples/channel", "N sets to save": Value Change {
        # "So that if 'Save ave N' is updated, the AOD scanning code updates too."
        n1173 = event-data() -> ()  [unwired: 6 out]
        n1174 = local read "AI Count (ticks)"() -> (w4511:u32)
        n1175 = Boolean To (0,1)(Boolean="Sets to FIFO (Traps)") -> (0, 1=w4521:cluster{"Set 1":i16, "Set 2":i16, "Set 3":i16})
        n1176 = xnode "Read/Write Control"("FPGA VI Reference In"=w4531, "error in"=w4529, "ai count"=w4511, "AI1 Sets to FIFO"="Sets to FIFO (Traps)", "N of AI1 Int Acq Sets"="N Acq Sets (Traps + Fl.)") -> ("error out"=w4530:errorcluster)  [unwired: 1 out]
        n1177 = Cluster To Array(cluster=w4521) -> (array=w4520:i16[])
        n1178 = To Unsigned Long Integer(number=w4520) -> (unsigned 32bit integer=w4500:u32[])
        n1179 = local read "Scan steps (AOD)"() -> (w4522:u64)
        n1180 = Multiply(x=w4511, y="N Acq Sets (Traps + Fl.)") -> (x*y=w4509:u32)
        n1181 = Divide(x=40000000.0, y=w4511) -> (x/y=w4503:dbl)
        "AI rate (Hz)" <- w4503
        "Ave. Rate (Hz)" <- w4503
        n1182 = Add Array Elements(numeric array=w4500) -> (sum=w4512:u32)
        "Trap Sets" <- w4512
        n1183 = Reciprocal(x=w4503) -> (1/x=→"Ave. Period (s)":dbl)
        n1184 = property on="Scan steps (AOD)" class="DigNum (strict)"("Val(Sgnl)"=w4522) -> ()  [unwired: 2 in, 2 out]
        n1185 = Divide(x=w4503, y="N Acq Sets (Traps + Fl.)") -> (x/y=w4526:dbl)
        "Data Rate (Hz)" <- w4526
        n1186 = Reciprocal(x=w4526) -> (1/x=→"Data Period (s)":dbl)
        n1187 = local read "Save ave N"() -> (w4525:dbl)
        n1188 = Divide(x=w4526, y=w4525) -> (x/y=w4524:dbl)
        "Save Data Rate (Hz)" <- w4524
        n1189 = Reciprocal(x=w4524) -> (1/x=→"Save Data Period (s)":dbl)
        n1190 = Multiply(x=w4509, y="# Samples/trap") -> (x*y=w4507:u32)
        "Counts/DMA" <- w4507
        n1191 = property on="Trap Disp. Downsample" class="DigNum (strict)"("Maximum"="# Samples/trap") -> ()  [unwired: 2 in, 2 out]
        n1192 = Multiply(x=w4512, y="# Samples/trap") -> (x*y=w4501:u32)
        "# Samples/channel" <- w4501
        n1193 = Multiply(x=w4501, y=u32 8) -> (x*y=→"Trap AI Elements/DMA read":u32)
        n1194 = local read "APD Int. Count"() -> (w4508:u32)
        n1195 = Multiply(x=w4501, y=u32 3) -> (x*y=→"Trap Pos Elements/DMA read":u32)
        n1196 = Divide(x=w4507, y=w4508) -> (x/y=w4498:dbl)
        "APD Samples/FIFO Acq." <- w4498
        n1197 = Divide(x=w4507, y=40000000.0) -> (x/y=w4505:dbl)
        "DMA Update Period (s)" <- w4505
        n1198 = Multiply(x=2.0, y=w4498) -> (x*y=→"APD Elements/DMA read":dbl)
        n1199 = property on="APD Disp. Downsample" class="DigNum (strict)"("Maximum"=w4498) -> ()  [unwired: 2 in, 2 out]
        n1200 = local read "N sets to save"() -> (w4518:u32)
        n1201 = Multiply(x=w4505, y=w4518) -> (x*y=→"Total Time (s)":dbl)
        "FPGA Averaging" <- FALSE ("FPGA Averaging")
      }
      event "Rescale on Mean": Value Change {
        n1202 = event-data() -> ()  [unwired: 7 out]
        n1203 = And(x=FALSE, y="Rescale on Mean") -> (x .and. y?=w4618:bool)
        n1204 = local write "Rescale on Mean"(w4618) -> ()
        n1205 = local read "Bead Mean (nm)"() -> (w4623:dbl)
        n1206 = Add(x="Amplitude (nm)", y=w4623) -> (x+y=w4621:dbl)
        n1207 = Subtract(x=w4623, y="Amplitude (nm)") -> (x-y=w4620:dbl)
        n1208 = property on="Bead Separation" class="WFChart (strict)"("YScale.Minimum"=w4620) -> ()  [unwired: 2 in, 2 out]
        n1209 = property on="Bead Separation" class="WFChart (strict)"("YScale.Maximum"=w4621) -> ()  [unwired: 2 in, 2 out]
      }
      event "Detector Type": Value Change {
        n1210 = event-data() -> ()  [unwired: 7 out]
        n1211 = local read "AI labels"() -> (w4624:string[])
        n1212 = property on="High Res. Display" class="Ring (strict)"("Strings []"=w4624) -> ()  [unwired: 2 in, 2 out]
        n1213 = Build Array (concatenate)(w4624, "none") -> (w4625:string[])
        n1214 = property on="FFT 1 Choice 1" class="Ring (strict)"("Strings []"=w4625) -> ()  [unwired: 2 in, 2 out]
        n1215 = property on="FFT 1 Choice 2" class="Ring (strict)"("Strings []"=w4625) -> ()  [unwired: 2 in, 2 out]
        n1216 = property on="FFT 2 Choice 1" class="Ring (strict)"("Strings []"=w4625) -> ()  [unwired: 2 in, 2 out]
        n1217 = property on="FFT 2 Choice 2" class="Ring (strict)"("Strings []"=w4625) -> ()  [unwired: 2 in, 2 out]
        n1218 = Bundle("APD 1", "APD 2") -> (w4628:cluster{string, string})  [unwired: 1 out]
        n1219 = Cluster To Array(cluster=w4628) -> (array=w4626:string[])
        n1220 = Build Array (concatenate)(w4626, w4625) -> (w4630:string[])
        n1221 = Array Size(array=w4630) -> (size(s)=w4631:i32)
        n1222 = property on="Signals to Plot" class="LstBox (strict)"("Item Names"=w4630) -> ()  [unwired: 2 in, 2 out]
        n1223 = property on="Signals to Plot" class="LstBox (strict)"("Number of Rows"=w4631) -> ()  [unwired: 2 in, 2 out]
        n1224 = property on="All Signals" class="WFChart (strict)"("LegNumRows"=w4631) -> ()  [unwired: 2 in, 2 out]
      }
      event "Adjust Scale\nto Mean": Value Change {
        n1225 = event-data() -> ()  [unwired: 7 out]
        n1226 = local read "APD 1 Rate (Hz)"() -> (w4640:dbl)
        n1227 = Multiply(x=1000.0, y="Above (kHz)") -> (x*y=w4638:dbl)
        n1228 = Multiply(x=1000.0, y="Below (kHz)") -> (x*y=w4636:dbl)
        n1229 = Add(x=w4638, y=w4640) -> (x+y=w4633:dbl)
        n1230 = Subtract(x=w4640, y=w4636) -> (x-y=w4634:dbl)
        n1231 = property on="APD Chart" class="WFChart (strict)"("YScale.Minimum"=w4634) -> ()  [unwired: 2 in, 2 out]
        n1232 = property on="APD Chart" class="WFChart (strict)"("YScale.Maximum"=w4633) -> ()  [unwired: 2 in, 2 out]
      }
      event "Phase adj. (AI1)", "+ phase (AI1)", "- phase (AI1)": Value Change {
        n1233 = event-data() -> ()  [unwired: 7 out]
        n1234 = Negate(x="Phase adj. (AI1)") -> (-x=w4650:i16)
        n1235 = Select(t=w4650, s="- phase (AI1)", f="Phase adj. (AI1)") -> (s? t:f=w4649:i16)
        n1236 = xnode "Read/Write Control"("FPGA VI Reference In"=w4653, "error in"=w4652, "Phase count adjustment"=w4649) -> ("FPGA VI Reference Out"=w4648:T20, "error out"=w4647:errorcluster)
        n1237 = Or(x="- phase (AI1)", y="+ phase (AI1)") -> (x .or. y?=w4644:bool)
        n1238 = xnode "Read/Write Control"("FPGA VI Reference In"=w4648, "error in"=w4647, "+ phase"=w4644) -> ("error out"=w4643:errorcluster)  [unwired: 1 out]
      }
      event "Signals to Plot": Double Click {
        w4731 = u32 9868950 ("Color Box")
        n1239 = event-data() -> ("Row"=w4733:i32)  [unwired: 9 out]
        n1240 = property on="All Signals" class="WFChart (strict)"("Active Plot"=w4733) -> (error out=w4744:errorcluster)  [unwired: 2 in, 1 out]
        n1241 = property on="All Signals" class="WFChart (strict)" props=["Plot", "Visible?", "Plot", "Plot Color"](error in=w4744) -> (error out=w4743:errorcluster, "Plot.Visible?"=w4742:bool)  [unwired: 1 in, 2 out]
        n1242 = Select(t=FALSE ("Plot.Visible"), s=w4742, f=TRUE ("Plot.Visible")) -> (s? t:f=w4737:bool)
        n1243 = property on="All Signals" class="WFChart (strict)"(error in=w4743, "Plot.Visible?"=w4737) -> (error out=w4739:errorcluster)  [unwired: 1 in, 1 out]
        n1244 = property on="All Signals" class="WFChart (strict)"(error in=w4739) -> (error out=w4734:errorcluster, "Plot.Plot Color"=w4738:u32)  [unwired: 1 in, 1 out]
        n1245 = property on="Signals to Plot" class="LstBox (strict)"(error in=w4734, "Active Row"=w4733) -> (error out=w4732:errorcluster)  [unwired: 1 in, 1 out]
        n1246 = Select(t=w4738, s=w4737, f=u32 0) -> (s? t:f=w4735:u32)
        n1247 = property on="Signals to Plot" class="LstBox (strict)"(error in=w4732, "CellFontColor"=w4735, "SelColor"=w4731, "CellBG"=w4731, "CellFontSize"=u32 20 ("Active Row:Cell Font:Size"), "CellFontBold"=TRUE ("Active Row:Cell Font:Bold")) -> ()  [unwired: 1 in, 2 out]
      }
      event "BD 1 Frequency 1 (MHz)", "BD 1 Frequency 2 (MHz)", "BD 1 Frequency 3 (MHz)", "BD 2 Frequency 1 (MHz)", "BD 2 Frequency 2 (MHz)", "BD 2 Frequency 3 (MHz)", "Trap Delta (MHz)": Value Change {
        # "anytime one of the frequencies is changed, write it to the RF board UNLESS Set 1 is being oscillated. The oscillation\nscript writes the frequencies to the RF board."
        n1248 = event-data() -> ("CtlRef"=w4747:refnum<vi>)  [unwired: 6 out]